vi "Experiment_UNKNOWN_IMPEDANCE.vi"() -> ()   [LabVIEW 2009]
uses:
  <vilib>/imath/engines/lvmath2/RunTimeEngine/ErrorHandling/NIMS_Finalize Error.vi
  <vilib>/imath/engines/lvmath2/RunTimeEngine/Parser/MC_Version.vi
  <vilib>/imath/engines/lvmath2/RunTimeEngine/NodeEndStatement/NIMS_NodeEndStatement_Output.vi
  <instcachedir>/0/NIMS_NodeEndStatement_Output_B70DDD75627E4997AAE11E9955EDAA25.lvgen/NIMS_NodeEndStatement_Output_B70DDD75627E4997AAE11E9955EDAA25_002.vi
  <instcachedir>/0/NIMS_NodeEndStatement_Output_B70DDD75627E4997AAE11E9955EDAA25.lvgen/NIMS_NodeEndStatement_Output_B70DDD75627E4997AAE11E9955EDAA25_003.vi
  <vilib>/imath/engines/lvmath/Functions/Error Handling/MergeErrorsWrapper.vi
  <instcachedir>/0/NIMS_NodeEndStatement_Output_B70DDD75627E4997AAE11E9955EDAA25.lvgen/NIMS_NodeEndStatement_Output_B70DDD75627E4997AAE11E9955EDAA25_000.vi
  <vilib>/imath/engines/lvmath2/RunTimeEngine/Managers/WorkSpace/UID Generator.vi
  <vilib>/imath/engines/lvmath/Functions/Error Handling/error.ctl
  <instcachedir>/0/NIMS_NodeEndStatement_Output_B70DDD75627E4997AAE11E9955EDAA25.lvgen/NIMS_NodeEndStatement_Output_B70DDD75627E4997AAE11E9955EDAA25_001.vi
  <vilib>/imath/engines/lvmath2/RunTimeEngine/Managers/SymbolTable/Clear UID.vi
  <vilib>/imath/engines/lvmath2/RunTimeEngine/VariableToken/NIMS_VariableToken_CondDefined.vi
  <instcachedir>/0/NIMS_VariableToken_CondDefined_5641E79000FB4D628475532441475385.lvgen/NIMS_VariableToken_CondDefined_5641E79000FB4D628475532441475385_002.vi
  <vilib>/imath/engines/lvmath/Functions/Error Handling/MC_Mask_Errors.vi
  <vilib>/imath/engines/lvmath2/RunTimeEngine/BuiltInFunctions/rem/NIMS_rem_no checks.vi
  <instcachedir>/0/NIMS_rem_no checks_4CC9B305AB7E42EF90AFC4973FB32F8D.lvgen/NIMS_rem_no checks_4CC9B305AB7E42EF90AFC4973FB32F8D_000.vi
  <vilib>/imath/engines/lvmath2/RunTimeEngine/BuiltInFunctions/uint32/NIMS_uint32(real).vi
  <instcachedir>/0/NIMS_uint32(real)_FDC83D68D45943DDB8F3F934FF8A712F.lvgen/NIMS_uint32(real)_FDC83D68D45943DDB8F3F934FF8A712F_000.vi
  <vilib>/imath/engines/lvmath2/RunTimeEngine/BuiltInFunctions/double/NIMS_double.vi
  <instcachedir>/0/NIMS_double_2CE444F3CE4146B199A482FE12545E45.lvgen/NIMS_double_2CE444F3CE4146B199A482FE12545E45_000.vi
  <vilib>/imath/engines/lvmath2/RunTimeEngine/RangeToken/NIMS_Range.vi
  <instcachedir>/0/NIMS_Range_6D647EC16A744C98B5DE1D649A2D648D.lvgen/NIMS_Range_6D647EC16A744C98B5DE1D649A2D648D_001.vi
  <vilib>/imath/engines/lvmath2/RunTimeEngine/BuiltInFunctions/length/NIMS_length(GV).vi
  <instcachedir>/0/NIMS_length(GV)_7D6E94E728E145E68721C53861296D96.lvgen/NIMS_length(GV)_7D6E94E728E145E68721C53861296D96_000.vi
  <instcachedir>/0/NIMS_Range_6D647EC16A744C98B5DE1D649A2D648D.lvgen/NIMS_Range_6D647EC16A744C98B5DE1D649A2D648D_000.vi
  <vilib>/imathl/engines/lvmath/Functions/Error Handling/Create Error.vi
  <vilib>/imath/engines/lvmath2/RunTimeEngine/ReplaceToken/NIMS_Replace - V(S)=S.vi
  <instcachedir>/0/NIMS_Replace - V(S)=S_670A9E0533664C1D848C8E58B3321B6A.lvgen/NIMS_Replace - V(S)=S_670A9E0533664C1D848C8E58B3321B6A_001.vi
  <vilib>/imath/engines/lvmath2/RunTimeEngine/ReplaceToken/NIMS_Replace - Size Check _(_)=S.vi
  <instcachedir>/0/NIMS_Replace - Size Check _(_)=S_8596181D73404097BAB9CBB006194BB0.lvgen/NIMS_Replace - Size Check _(_)=S_8596181D73404097BAB9CBB006194BB0_002.vi
  <vilib>/imath/engines/lvmath2/RunTimeEngine/ReplaceToken/NIMS_Replace - Check Linear.vi
  <instcachedir>/0/NIMS_Replace - Check Linear_9243CBB174894FF6977027453DA6955E.lvgen/NIMS_Replace - Check Linear_9243CBB174894FF6977027453DA6955E_002.vi
  <vilib>/imath/engines/lvmath2/RunTimeEngine/VariableToken/NIMS_VariableToken_CondDefinedDefinedByReplace.vi
  <instcachedir>/0/NIMS_VariableToken_CondDefinedDefinedByReplace_D162CFFC24174562A9FEA619A91E1A56.lvgen/NIMS_VariableToken_CondDefinedDefinedByReplace_D162CFFC24174562A9FEA619A91E1A56_002.vi
  <vilib>/imath/engines/lvmath2/RunTimeEngine/CommandStatement/MC_CommandStatement_break.vi
  <vilib>/imath/engines/lvmath2/RunTimeEngine/LocalVariableDefStatement/MC_LocalVariableDefStatement_Display.vi
  <vilib>/imath/engines/lvmath2/RunTimeEngine/RunTimeType/NIMS_RunTimeType_From StrictType (excl LVString).vi
  <vilib>/imath/engines/lvmath2/RunTimeEngine/ArithmeticOperatorToken/NIMS_ArithmeticOperator_times.vi
  <instcachedir>/0/NIMS_ArithmeticOperator_times_3987BC660D7947CD8628C10658A43225.lvgen/NIMS_ArithmeticOperator_times_3987BC660D7947CD8628C10658A43225_001.vi
  <instcachedir>/0/NIMS_ArithmeticOperator_times_3987BC660D7947CD8628C10658A43225.lvgen/NIMS_ArithmeticOperator_times_3987BC660D7947CD8628C10658A43225_000.vi
  <vilib>/imath/engines/lvmath2/RunTimeEngine/VariableToken/Read/NIMS_Get Elements - RV(_) - Check.vi
  <instcachedir>/0/NIMS_Get Elements - RV(_) - Check_60F12861D0564803969A5D0D0D1716CD.lvgen/NIMS_Get Elements - RV(_) - Check_60F12861D0564803969A5D0D0D1716CD_001.vi
  <instcachedir>/0/NIMS_VariableToken_CondDefined_5641E79000FB4D628475532441475385.lvgen/NIMS_VariableToken_CondDefined_5641E79000FB4D628475532441475385_001.vi
  <vilib>/imath/engines/lvmath2/RunTimeEngine/BuiltInFunctions/abs/NIMS_abs(signed).vi
  <instcachedir>/0/NIMS_abs(signed)_C4FCB8E6058B49B797C7C8D53CA5F6EC.lvgen/NIMS_abs(signed)_C4FCB8E6058B49B797C7C8D53CA5F6EC_000.vi
  <instcachedir>/0/NIMS_Replace - V(S)=S_670A9E0533664C1D848C8E58B3321B6A.lvgen/NIMS_Replace - V(S)=S_670A9E0533664C1D848C8E58B3321B6A_000.vi
  <instcachedir>/0/NIMS_Replace - Size Check _(_)=S_8596181D73404097BAB9CBB006194BB0.lvgen/NIMS_Replace - Size Check _(_)=S_8596181D73404097BAB9CBB006194BB0_001.vi
  <instcachedir>/0/NIMS_Replace - Check Linear_9243CBB174894FF6977027453DA6955E.lvgen/NIMS_Replace - Check Linear_9243CBB174894FF6977027453DA6955E_001.vi
  <instcachedir>/0/NIMS_VariableToken_CondDefinedDefinedByReplace_D162CFFC24174562A9FEA619A91E1A56.lvgen/NIMS_VariableToken_CondDefinedDefinedByReplace_D162CFFC24174562A9FEA619A91E1A56_001.vi
  <instcachedir>/0/NIMS_Replace - V(S)=S_670A9E0533664C1D848C8E58B3321B6A.lvgen/NIMS_Replace - V(S)=S_670A9E0533664C1D848C8E58B3321B6A_002.vi
  <instcachedir>/0/NIMS_Replace - Size Check _(_)=S_8596181D73404097BAB9CBB006194BB0.lvgen/NIMS_Replace - Size Check _(_)=S_8596181D73404097BAB9CBB006194BB0_003.vi
  <instcachedir>/0/NIMS_Replace - Check Linear_9243CBB174894FF6977027453DA6955E.lvgen/NIMS_Replace - Check Linear_9243CBB174894FF6977027453DA6955E_003.vi
  <instcachedir>/0/NIMS_VariableToken_CondDefinedDefinedByReplace_D162CFFC24174562A9FEA619A91E1A56.lvgen/NIMS_VariableToken_CondDefinedDefinedByReplace_D162CFFC24174562A9FEA619A91E1A56_003.vi
  <vilib>/imath/engines/lvmath2/RunTimeEngine/BuiltInFunctions/imag/NIMS_imag(Complex).vi
  <instcachedir>/0/NIMS_imag(Complex)_D35A2F120E254B34824E500A22AD8EA0.lvgen/NIMS_imag(Complex)_D35A2F120E254B34824E500A22AD8EA0_000.vi
  <vilib>/imath/engines/lvmath2/RunTimeEngine/Managers/SymbolTable/NIMS_WorkSpace.lvlib
panel:
  out "error out":errorcluster
  in  "HELP FOR VSWR":bool
  out "error out":errorcluster
  out "?":errorcluster
  in  "VSWR Value of Unknown Impedance":bool
  out "?":errorcluster
  out "VSWR Meter":dbl(knob) caption="Meter" scale=500.0..1.0 scale format="%#_10g"
  in  "?":enum32{"LOADS"}(tab)
  in  "Type of Loads":T1(radio)
  out "Resistance 2":dbl
  out "Reactance":dbl
  in  "Resistance":dbl(slide) scale=0.0..1000.0
  in  "Reluctance":dbl(slide) scale=0.0..1000.0
  out "?":errorcluster
  in  "HELP FOR LOADS":bool
  out "error out":errorcluster
  in  "?":enum32{"SLOTTED LINE(VOLTAGE)"}(tab)
  out "?":dbl[](graph)
  in  "Slide":dbl(slide) scale=0.0..0.3
  out "Voltage":dbl
  out "Distance(Meter)":dbl
  out "Characteristic Impedance":dbl
  in  "Short Circuited              Load":bool
  out "?":errorcluster
  in  "First Minima from Load(Unknown Impedance)":bool
  out "?":dbl
  in  "First Minima from Load(Short Circuited)":bool
  in  "Second Minima from Load(Short Circuited)":bool
  out "?":dbl
  in  "HELP FOR SLOTTED LINE":bool
  out "?":dbl
  in  "?":enum32{"ATTENUATOR"}(tab)
  out "?":dbl[](graph)
  in  "Set the value of attenuation in dB":dbl(slide) scale=0.0..100.0
  out "?":errorcluster
  in  "HELP FOR ATTENUATOR":bool
  out "error out":errorcluster
  in  "?":enum32{"ISOLATOR"}(tab)
  out "?":dbl[](graph)
  in  "?":bool
  out "?":errorcluster
  in  "HELP FOR ISOLATOR":bool
  out "error out":errorcluster
  in  "?":enum32{"MODULATOR"}(tab)
  out "?":dbl[](graph)
  in  "Modulating Frequency(KHz)":dbl(slide) scale=0.5..1.5
  out "?":errorcluster
  in  "HELP FOR MODULATOR":bool
  out "error out":errorcluster
  in  "?":enum32{"SOURCE"}(tab)
  out "?":dbl[](graph)
  in  "Frequency of carrier wave(GHz)":dbl(slide) scale=8.0..15.0
  in  "Voltage 3":dbl(knob) scale=0.0..20.0 scale format="%#_10g"
  out "?":errorcluster
  in  "HELP FOR SOURCE":bool
  out "error out":errorcluster
  out "?":errorcluster
  out "Reactance of Unknown Impedance":dbl
  out "Resistance of Unknown Impedance":dbl
  in  "Value of Unknown Impedance":bool
  # "Source"
  # "Variable Attenuator"
  # "Slotted Line"
  # "Coaxial to rectangular adapter"
  # "Variable load"
  # "Connecting waveguide"
  # "Connecting waveguide"
  # "Connecting waveguide"
  # "Isolator"
  # "Matched load"
  # "VSWR Meter"
  # "Backward Direction"
  # "Forward direction"
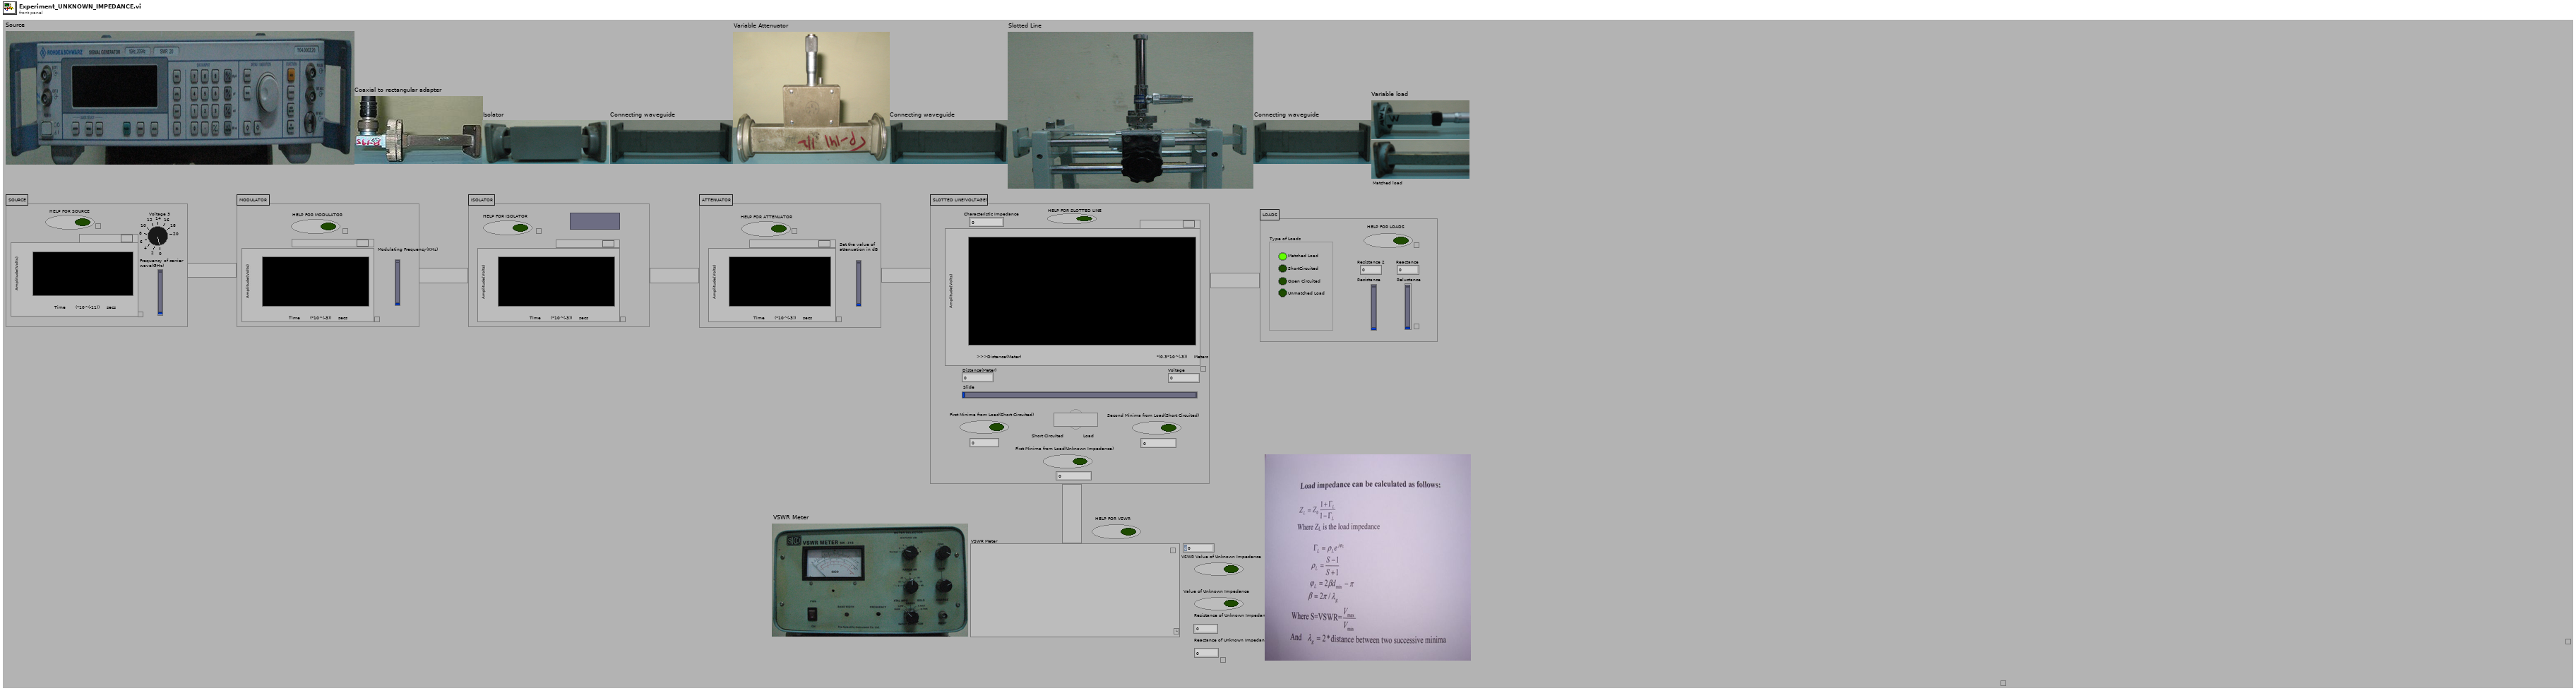
[diagram p1: front panel]
types:
  T1 = enum32{"Matched Load", "ShortCircuited", "Open Circuited", "Unmatched Load"}
  T2 = typedef "error.ctl" = enum16{"No Error", "Problem", "Unused002", "Incorrect number of parameters", "Function not defined for non-numeric types", "Unused005", "Function only defined for character arrays", "Function not defined for boolean, character, or single precision", "Function not defined for complex types", "Not a valid operation", "Inputs must be scalar", "Input matrices are not the same size", "Unused012", "Input matrices must be nonnegative integers of the same type", "Arguments must be non-negative integers less than bitmax", "Number to complement must be less than 2^N", "Bit to get is outside range", "Bit to set is outside range", "Input must be real type ", "At least one parameter must be scalar", "Unused020", "Function not defined for\nhigher dimensional matrices.", "Invalid attributes", "Wrong Type of Input Arguments", "Wrong Argument Option", "Unused025", "Indices must be real positive integers", "Unused027", "Number of elements must be the same for indices and values", "Unused029", "Cannot resize a 2D matrix with a linear index", "Unknown variable or symbol", "Indices out of range", "Empty matrix deletion can not be used with two indices", "Number of rows and columns must be the same for indices and values.", "Complex cannot be converted to Boolean", "Char cannot be converted to Boolean", "int64 cannot be converted to Boolean", "uint64 cannot be converted to Boolean", "Unused039", "Unused040", "All rows must have the same number of columns", "Incompatible types", "Invalid matrix dimensions", "Dimension must be 1 or 2", "Base must be an integer between 2 and 36", "Invalid input", "Square matrix required", "Function 'timerstart' must be called before 'timerstop'", "Arguments must be positive real", "Step must not be zero", "Wrong number of input arguments", "Wrong number of output arguments", "Unused053", "Input scalar must be >= 0", "Input scalar must be positive", "Input scalar must not be 0", "Input scalar must be in range [0,1]", "Unused058", "Input must be a vector", "Unused060", "Empty vector error", "All elements must be in domain [-1,1]", "All real elements of input vector must be >= 0", "All elements of input vector must be positive", "Values of input vectors are not compatible", "Unused066", "Input vector must be an increasing vector", "Unused068", "Unused069", "Lenths of two input vectors are not compatible", "Unused071", "Empty matrix error", "Unused073", "Unused074", "Unused075", "Unused076", "Unused077", "Size of input matrix is incompatible with input size", "Invalid format specifier", "Unused080", "Unused081", "Unused082", "Unused083", "Unused084", "Unused085", "RunTime: MathScript could not be compiled", "Unknown function", "Only scalars and strings supported", "Unused089", "Unused090", "Range is too large", "End used without variable", "Function not available (RTE)", "Custom user error", "Arguments must be integers less than bitmax", "Shared library not found", "Header file not found", "Shared library already loaded", "Shared library not loaded", "Shared library function not found", "Shared library string return problem", "Problem calling shared library function", "Problem loading shared library from OS", "Problem parsing shared library header file", "Shared library incompatible types", "Shared library unsupported return type", "Shared library function not exported", "Shared library unsupported input type", "Problem unloading shared library from OS", "Function only available from UI", "Invalid function specified in argument", "An internal error has occurred", "Invalid object", "Invalid property", "Read-only property", "A break command has occurred", "A continue command has occurred", "A return command has occurred", "ode: times parameter invalid", "Unused120", "Function not found in file", "Reserved keyword cannot be defined as variable", "Reserved keyword cannot be defined as a function or script", "Arguments must be string literals", "Function not supported on this platform", "All columns must have the same number of rows", "Function ignored in RTE warning", "Cannot use : as a parameter that is not a variable", "Output can't be coerced to requested type", "Function not supported on current target", "Variable dependent on an unwired function input", "Unused132", "Unused133", "Unused134", "Unused135", "Unused136", "Unused137", "Unused138", "Unused139", "Unused140", "Unused141", "Unused142", "Unused143", "Unused144", "Unused145", "Unused146", "MathScript parser DLL missing", "MathScript requires LabVIEW Full", "MathScript license is invalid or missing"}
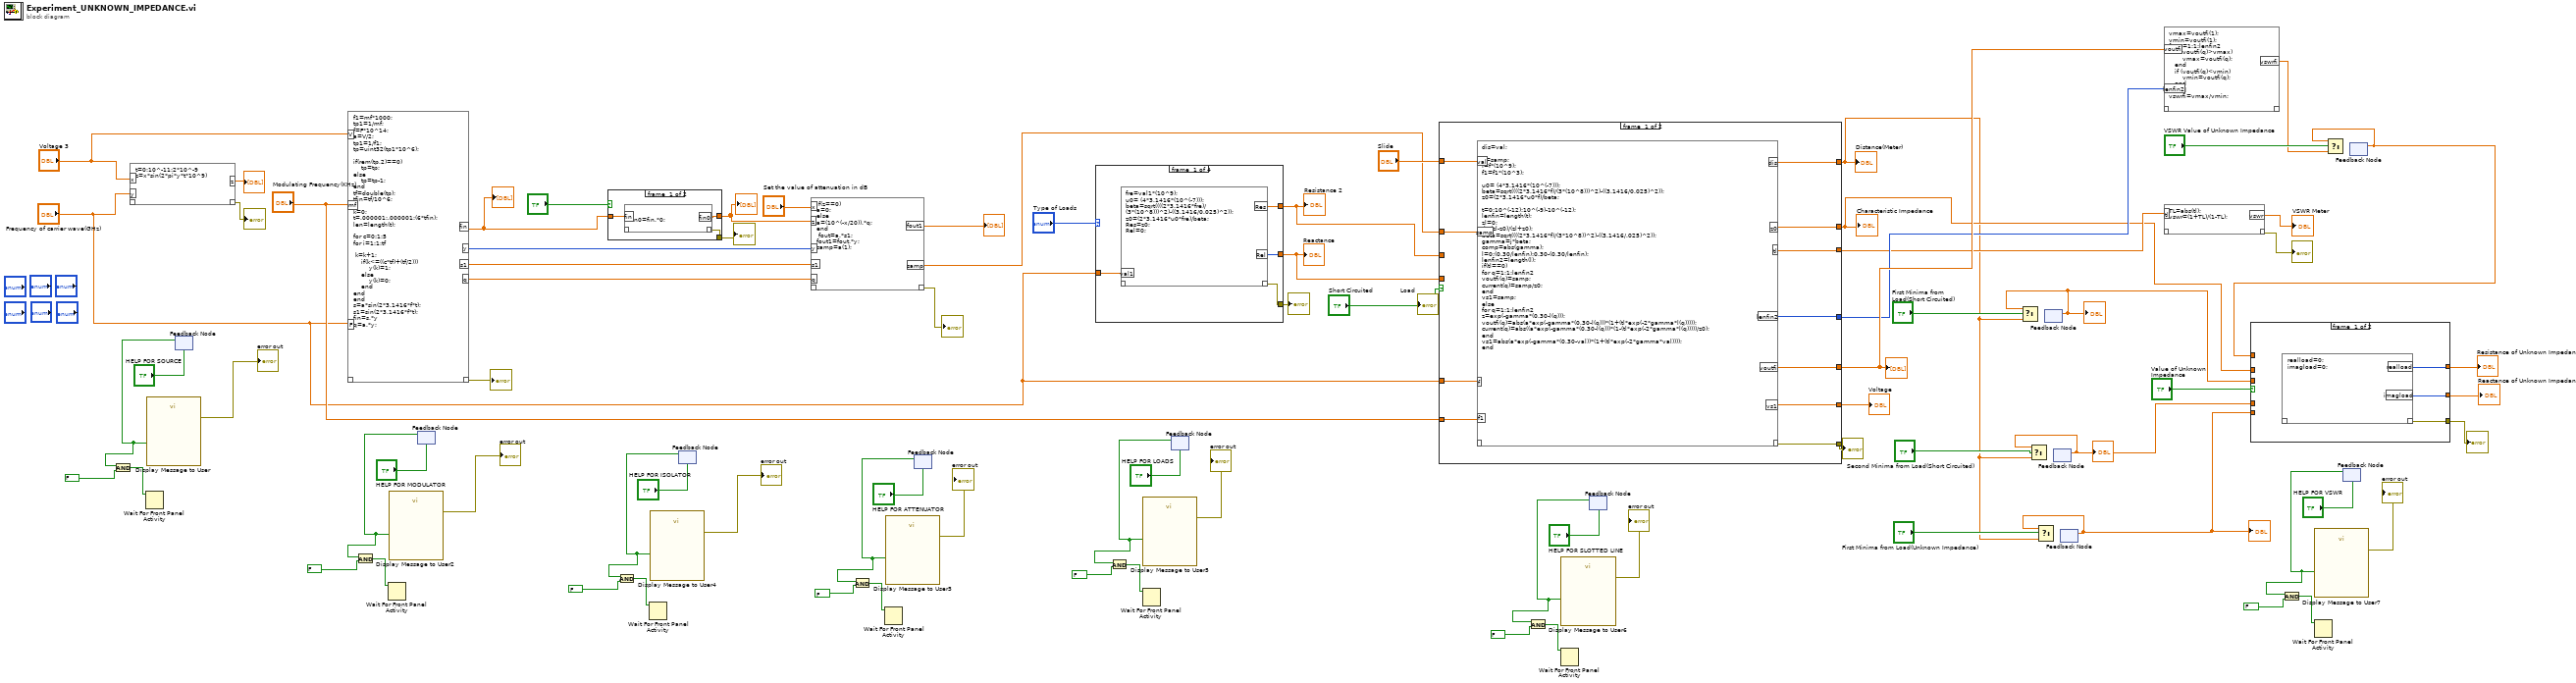
[diagram p0: block diagram]
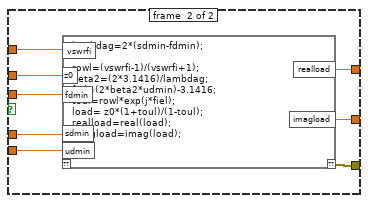
[diagram p2: hidden frame]
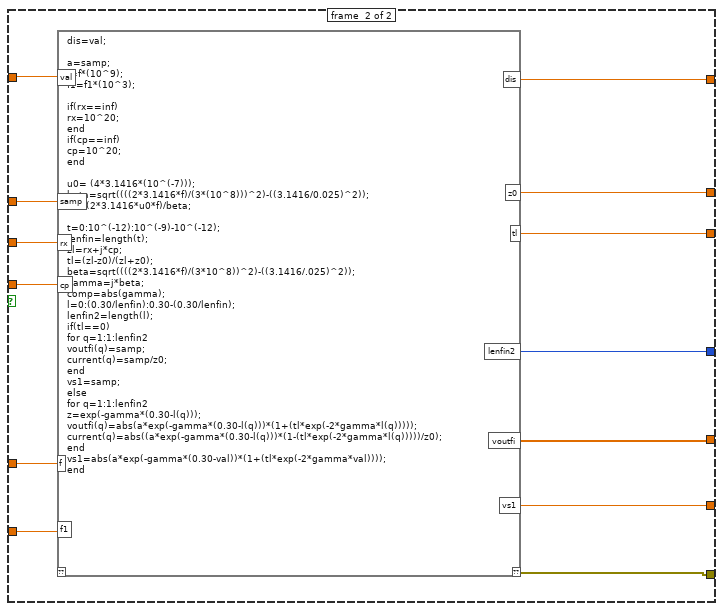
[diagram p3: hidden frame]
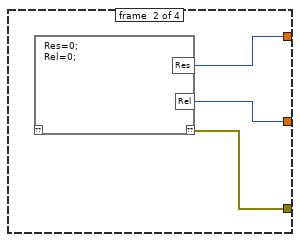
[diagram p4: hidden frame]
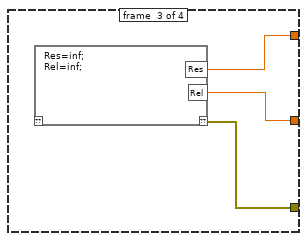
[diagram p5: hidden frame]
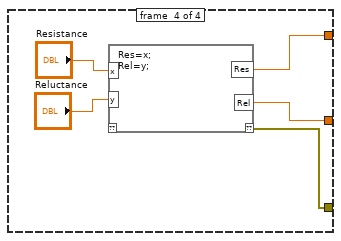
[diagram p6: hidden frame]
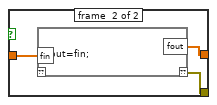
[diagram p7: hidden frame]
diagram:
  n1 = mathscript code="t=0:10^-11:2*10^-9\nz=x*sin(2*pi*y*t*10^9)"("x"="Voltage 3", "y"="Frequency of carrier wave(GHz)") -> ("??"=→"?":errorcluster, "z"=→"?":dbl[])  [unwired: 1 in]
  n2 = feedback #1("HELP FOR SOURCE") -> (w75:bool)
  n3 = And(x=w75, y=FALSE) -> (x .and. y?=w73:bool)
  n4 = Wait For Front Panel Activity(3:w73) -> ()  [unwired: 3 out]
  n5 = call "Display Message to User"("Enable"=w75) -> ("error out"=→"error out":errorcluster, "CLOSE"=w77:bool)  [unwired: 2 in, 7 out]
  n6 = mathscript code="f1=mf*1000;\ntp1=1/mf;\nf=F*10^14;\na=V/2;\ntp1=1/f1;\ntp=uint32(tp1*10^6);\n\nif(rem(tp,2)==0)\n    tp=tp;\nelse\n    tp=tp-1;\nend\ntf=double(tp);\ntfin=tf/10^6;\n\nk=0;\nt=.000001:.000001:(6*tfin);\nlen=length(t);\n\nfor c=0:1:5\nfor i=1:1:tf\n  \n k=k+1;\n    if(k<=((c*tf)+(tf/2)))\n        y(k)=1;\n    else\n        y(k)=0;\n    end\nend\nend\ns=a*sin(2*3.1416*f*t);\ns1=sin(2*3.1416*f*t);\nfin=s.*y\nq=a.*y;"("V"="Voltage 3", "mf"="Modulating Frequency(KHz)", "F"="Frequency of carrier wave(GHz)") -> ("??"=→"?":errorcluster, "fin"=w31:dbl[], "y"=w27:i32[], "s1"=w26:dbl[], "q"=w25:dbl[])  [unwired: 1 in]
  "?" <- w31
  n7 = feedback #2("HELP FOR MODULATOR") -> (w69:bool)
  n8 = And(x=w69, y=FALSE) -> (x .and. y?=w67:bool)
  n9 = Wait For Front Panel Activity(3:w67) -> ()  [unwired: 3 out]
  n10 = call "Display Message to User2"("Enable"=w69) -> ("error out"=→"error out":errorcluster, "CLOSE"=w71:bool)  [unwired: 2 in, 7 out]
  n11 = case shown="False" "?" {
    tunnel: w31 -> [w94 w115]
    tunnel: [w92 w114] -> w87
    tunnel: [w93 w113] -> w28
    frame #0 {
      n12 = mathscript code="fin0=fin.*0;"("fin"=w94) -> ("??"=w92:errorcluster, "fin0"=w93:dbl[])  [unwired: 1 in]
    }
    frame #1 {
      n13 = mathscript code="fout=fin;"("fin"=w115) -> ("??"=w114:errorcluster, "fout"=w113:dbl[])  [unwired: 1 in]
    }
  }
  "?" <- w28
  "?" <- w87
  n14 = feedback #3("HELP FOR ISOLATOR") -> (w57:bool)
  n15 = And(x=w57, y=FALSE) -> (x .and. y?=w55:bool)
  n16 = Wait For Front Panel Activity(3:w55) -> ()  [unwired: 3 out]
  n17 = call "Display Message to User4"("Enable"=w57) -> ("error out"=→"error out":errorcluster, "CLOSE"=w59:bool)  [unwired: 2 in, 7 out]
  n18 = mathscript code="if(z==0)\na=0; \nelse\na=(10^(-x/20)).*q;\nend\n fout=a.*s1;\nfout1=fout.*y;\nsamp=a(1);"("x"="Set the value of attenuation in dB", "z"=w28, "y"=w27, "s1"=w26, "q"=w25) -> ("??"=→"?":errorcluster, "fout1"=→"?":dbl[], "samp"=w22:dbl)  [unwired: 1 in]
  n19 = feedback #4("HELP FOR ATTENUATOR") -> (w63:bool)
  n20 = And(x=w63, y=FALSE) -> (x .and. y?=w61:bool)
  n21 = Wait For Front Panel Activity(3:w61) -> ()  [unwired: 3 out]
  n22 = call "Display Message to User3"("Enable"=w63) -> ("error out"=→"error out":errorcluster, "CLOSE"=w65:bool)  [unwired: 2 in, 7 out]
  n23 = case shown="\"Unmatched Load\"" "Type of Loads" {
    tunnel: "Frequency of carrier wave(GHz)" -> [w135 _ _ _]
    tunnel: [w132 w221 w248 w274] -> w89
    tunnel: [w133 w220 w247 w273] -> w88
    tunnel: [w134 w222 w246 w272] -> w86
    frame #0 {
      n24 = mathscript code="fre=val1*(10^9);\nu0= (4*3.1416*(10^(-7)));\nbeta=sqrt((((2*3.1416*fre)/(3*(10^8)))^2)-((3.1416/0.025)^2));\nz0=(2*3.1416*u0*fre)/beta;\nRes=z0;\nRel=0;"("val1"=w135) -> ("??"=w134:errorcluster, "Res"=w132:cdb, "Rel"=w133:i32)  [unwired: 1 in]
    }
    frame #1 {
      n25 = mathscript code="Res=0;\nRel=0;"() -> ("??"=w222:errorcluster, "Res"=w221:i32, "Rel"=w220:i32)  [unwired: 1 in]
    }
    frame #2 {
      n26 = mathscript code="Res=inf;\nRel=inf;"() -> ("??"=w246:errorcluster, "Res"=w248:dbl, "Rel"=w247:dbl)  [unwired: 1 in]
    }
    frame #3 {
      n27 = mathscript code="Res=x;\nRel=y;"("x"="Resistance", "y"="Reluctance") -> ("??"=w272:errorcluster, "Res"=w274:dbl, "Rel"=w273:dbl)  [unwired: 1 in]
    }
  }
  "Resistance 2" <- w89
  "Reactance" <- w88
  "?" <- w86
  n28 = feedback #5("HELP FOR LOADS") -> (w51:bool)
  n29 = And(x=w51, y=FALSE) -> (x .and. y?=w49:bool)
  n30 = Wait For Front Panel Activity(3:w49) -> ()  [unwired: 3 out]
  n31 = call "Display Message to User5"("Enable"=w51) -> ("error out"=→"error out":errorcluster, "CLOSE"=w53:bool)  [unwired: 2 in, 7 out]
  n32 = case shown="True" "Short Circuited              Load" {
    tunnel: w89 -> [_ w893]
    tunnel: w88 -> [_ w892]
    tunnel: [w309 w888] -> w15
    tunnel: "Frequency of carrier wave(GHz)" -> [w312 w891]
    tunnel: "Modulating Frequency(KHz)" -> [w311 w890]
    tunnel: w22 -> [w313 w894]
    tunnel: [w304 w883] -> w85
    tunnel: [w306 w885] -> w21
    tunnel: [w308 w887] -> w19
    tunnel: "Slide" -> [w314 w895]
    tunnel: [w305 w884] -> w82
    tunnel: [w310 w889] -> w7
    tunnel: [w307 w886] -> w20
    frame #0 {
      n33 = mathscript code="dis=val;\n\na=samp;\nf=f*(10^9);\nf1=f1*(10^3);\n\nu0= (4*3.1416*(10^(-7)));\nbeta=sqrt((((2*3.1416*f)/(3*(10^8)))^2)-((3.1416/0.025)^2));\nz0=(2*3.1416*u0*f)/beta;\n\nt=0:10^(-12):10^(-9)-10^(-12);\nlenfin=length(t);\nzl=0;\ntl=(zl-z0)/(zl+z0);\nbeta=sqrt((((2*3.1416*f)/(3*10^8))^2)-((3.1416/.025)^2));\ngamma=j*beta;\ncomp=abs(gamma);\nl=0:(0.30/lenfin):0.30-(0.30/lenfin);\nlenfin2=length(l);\nif(tl==0)\nfor q=1:1:lenfin2\nvoutfi(q)=samp;\ncurrent(q)=samp/z0;\nend\nvs1=samp;\nelse\nfor q=1:1:lenfin2\nz=exp(-gamma*(0.30-l(q)));\nvoutfi(q)=abs(a*exp(-gamma*(0.30-l(q)))*(1+(tl*exp(-2*gamma*l(q)))));\ncurrent(q)=abs((a*exp(-gamma*(0.30-l(q)))*(1-(tl*exp(-2*gamma*l(q)))))/z0);\nend\nvs1=abs(a*exp(-gamma*(0.30-val))*(1+(tl*exp(-2*gamma*val))));\nend"("val"=w314, "samp"=w313, "f"=w312, "f1"=w311) -> ("??"=w304:errorcluster, "dis"=w310:dbl, "z0"=w309:cdb, "tl"=w308:cdb, "lenfin2"=w307:i32, "voutfi"=w306:dbl[], "vs1"=w305:dbl)  [unwired: 1 in]
    }
    frame #1 {
      n34 = mathscript code="dis=val;\n\na=samp;\nf=f*(10^9);\nf1=f1*(10^3);\n\nif(rx==inf)\nrx=10^20;\nend\nif(cp==inf)\ncp=10^20;\nend\n\nu0= (4*3.1416*(10^(-7)));\nbeta=sqrt((((2*3.1416*f)/(3*(10^8)))^2)-((3.1416/0.025)^2));\nz0=(2*3.1416*u0*f)/beta;\n\nt=0:10^(-12):10^(-9)-10^(-12);\nlenfin=length(t);\nzl=rx+j*cp;\ntl=(zl-z0)/(zl+z0);\nbeta=sqrt((((2*3.1416*f)/(3*10^8))^2)-((3.1416/.025)^2));\ngamma=j*beta;\ncomp=abs(gamma);\nl=0:(0.30/lenfin):0.30-(0.30/lenfin);\nlenfin2=length(l);\nif(tl==0)\nfor q=1:1:lenfin2\nvoutfi(q)=samp;\ncurrent(q)=samp/z0;\nend\nvs1=samp;\nelse\nfor q=1:1:lenfin2\nz=exp(-gamma*(0.30-l(q)));\nvoutfi(q)=abs(a*exp(-gamma*(0.30-l(q)))*(1+(tl*exp(-2*gamma*l(q)))));\ncurrent(q)=abs((a*exp(-gamma*(0.30-l(q)))*(1-(tl*exp(-2*gamma*l(q)))))/z0);\nend\nvs1=abs(a*exp(-gamma*(0.30-val))*(1+(tl*exp(-2*gamma*val))));\nend"("val"=w895, "samp"=w894, "rx"=w893, "cp"=w892, "f"=w891, "f1"=w890) -> ("??"=w883:errorcluster, "dis"=w889:dbl, "z0"=w888:cdb, "tl"=w887:cdb, "lenfin2"=w886:i32, "voutfi"=w885:dbl[], "vs1"=w884:dbl)  [unwired: 1 in]
    }
  }
  "?" <- w21
  "Characteristic Impedance" <- w15
  "?" <- w85
  "Voltage" <- w82
  "Distance(Meter)" <- w7
  n35 = feedback #6("HELP FOR SLOTTED LINE") -> (w45:bool)
  n36 = And(x=w45, y=FALSE) -> (x .and. y?=w43:bool)
  n37 = Wait For Front Panel Activity(3:w43) -> ()  [unwired: 3 out]
  n38 = call "Display Message to User6"("Enable"=w45) -> ("error out"=→"error out":errorcluster, "CLOSE"=w47:bool)  [unwired: 2 in, 7 out]
  n39 = feedback #7() -> (w6:dbl)  [unwired: 1 in]
  "?" <- w6
  n40 = Select(t=w6, s="First Minima from Load(Short Circuited)", f=w7) -> (s? t:f=w13:dbl)
  n41 = feedback #8() -> (w11:dbl)  [unwired: 1 in]
  "?" <- w11
  n42 = Select(t=w11, s="Second Minima from Load(Short Circuited)", f=w7) -> (s? t:f=w12:dbl)
  n43 = feedback #9() -> (w5:dbl)  [unwired: 1 in]
  "?" <- w5
  n44 = Select(t=w5, s="First Minima from Load(Unknown Impedance)", f=w7) -> (s? t:f=w9:dbl)
  n45 = mathscript code="vmax=voutfi(1);\nvmin=voutfi(1);\nfor q=1:1:lenfin2\n   if (voutfi(q)>vmax)\n       vmax=voutfi(q);\n   end\n   if (voutfi(q)<vmin)\n       vmin=voutfi(q);\n   end\n   end\nvswrfi=vmax/vmin;"("lenfin2"=w20, "voutfi"=w21) -> ("vswrfi"=w2:dbl)  [unwired: 1 in, 1 out]
  n46 = mathscript code="TL=abs(tl);\nvswr=(1+TL)/(1-TL);"("tl"=w19) -> ("??"=→"?":errorcluster, "vswr"=→"VSWR Meter":dbl)  [unwired: 1 in]
  n47 = feedback #10("HELP FOR VSWR") -> (w39:bool)
  n48 = And(x=w39, y=FALSE) -> (x .and. y?=w37:bool)
  n49 = Wait For Front Panel Activity(3:w37) -> ()  [unwired: 3 out]
  n50 = call "Display Message to User7"("Enable"=w39) -> ("error out"=→"error out":errorcluster, "CLOSE"=w41:bool)  [unwired: 2 in, 7 out]
  n51 = feedback #11() -> (w1:dbl)  [unwired: 1 in]
  n52 = case shown="True" "Value of Unknown Impedance" {
    tunnel: [w1505 w1532] -> w81
    tunnel: [w1504 w1531] -> w80
    tunnel: w11 -> [_ w1534]
    tunnel: w5 -> [_ w1533]
    tunnel: w1 -> [_ w1536]
    tunnel: w15 -> [_ w1535]
    tunnel: [w1503 w1530] -> w16
    tunnel: w6 -> [_ w1529]
    frame #0 {
      n53 = mathscript code="realload=0;\nimagload=0;"() -> ("??"=w1503:errorcluster, "realload"=w1505:i32, "imagload"=w1504:i32)  [unwired: 1 in]
    }
    frame #1 {
      n54 = mathscript code="lambdag=2*(sdmin-fdmin);\n\nrowl=(vswrfi-1)/(vswrfi+1);\nbeta2=(2*3.1416)/lambdag;\nfiel=(2*beta2*udmin)-3.1416;\ntoul=rowl*exp(j*fiel);\nload= z0*(1+toul)/(1-toul);\nrealload=real(load);\nimagload=imag(load);"("vswrfi"=w1536, "z0"=w1535, "fdmin"=w1529, "sdmin"=w1534, "udmin"=w1533) -> ("??"=w1530:errorcluster, "realload"=w1532:dbl, "imagload"=w1531:dbl)  [unwired: 1 in]
    }
  }
  "Resistance of Unknown Impedance" <- w81
  "Reactance of Unknown Impedance" <- w80
  "?" <- w16
  n55 = Select(t=w1, s="VSWR Value of Unknown Impedance", f=w2) -> (s? t:f=w4:dbl)
